vi "MPS_main.vi"() -> ()   [LabVIEW 2021] (continued)
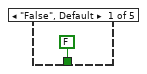
[diagram p2: hidden frame]
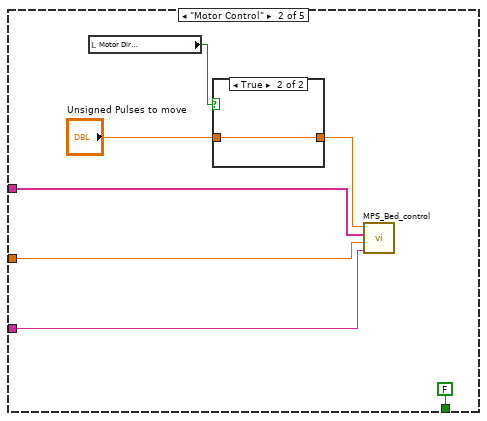
[diagram p3: hidden frame]
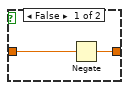
[diagram p4: hidden frame]
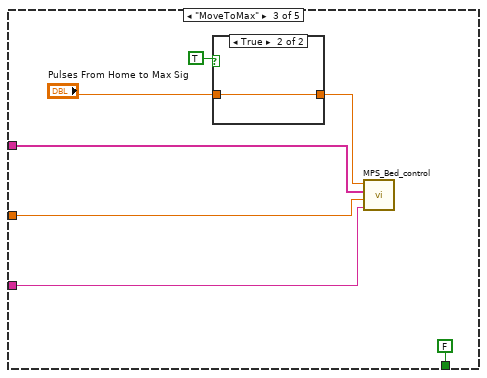
[diagram p5: hidden frame]
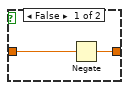
[diagram p6: hidden frame]
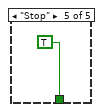
[diagram p7: hidden frame]
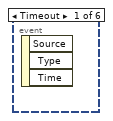
[diagram p8: hidden frame]
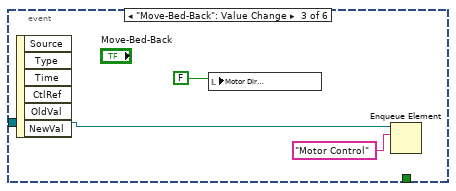
[diagram p9: hidden frame]
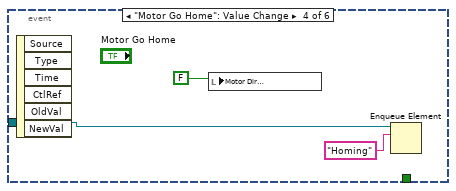
[diagram p10: hidden frame]
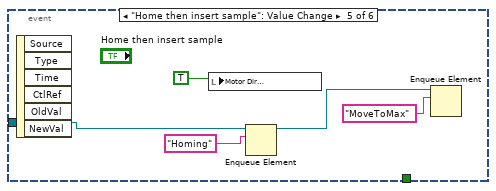
[diagram p11: hidden frame]
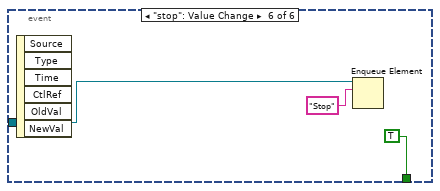
[diagram p12: hidden frame]
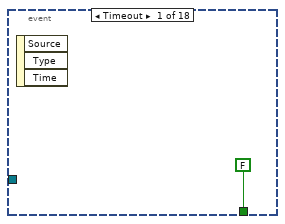
[diagram p13: hidden frame]
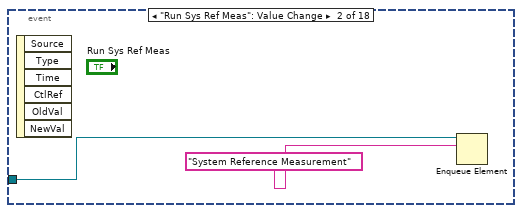
[diagram p14: hidden frame]
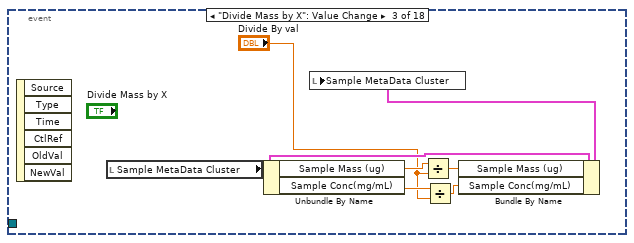
[diagram p15: hidden frame]
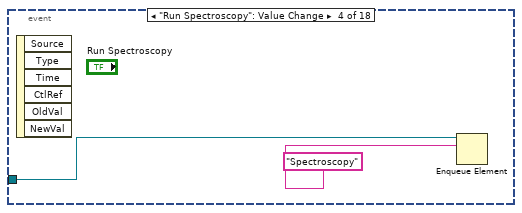
[diagram p16: hidden frame]
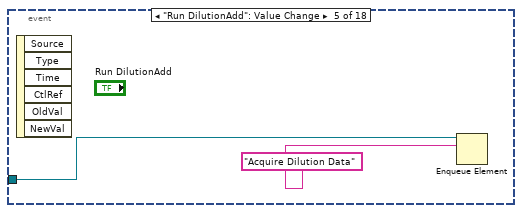
[diagram p17: hidden frame]
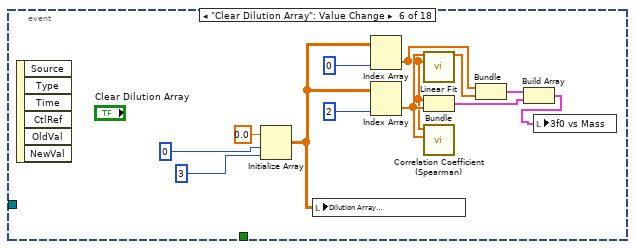
[diagram p18: hidden frame]
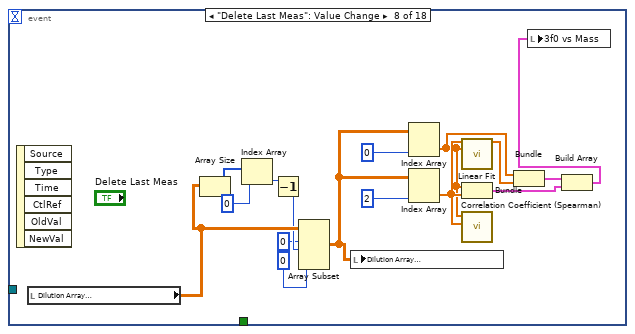
[diagram p19: hidden frame]
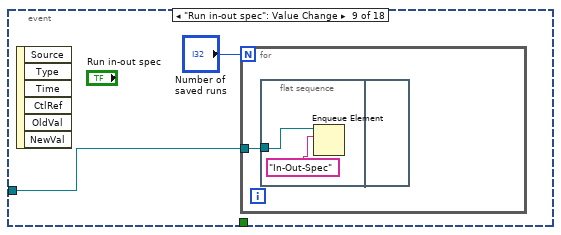
[diagram p20: hidden frame]
            n301 = global read "MPS_global_variables.vi" "Device Name"() -> (w392:tag)
            n302 = call "save_MPS_spectroscopy_hdf.vi"("file path"=w415, "Device Name"=w392, "Phase Rx over time"=w412, "Mag Rx over time"=w413, "TxRx_Params"=w414, "Rx_f0-f8 Units"=w408, "Time Domain Cluster"=w418, "Sample MetaData Cluster"=w399, "Study and Experiment Description"=w400, "Scanner Description"=w401, "Points from home to max"=w402) -> ()  [unwired: 5 in]
          }
        }
        n303 = call <vilib>:"Std Deviation and Variance.vi"("X"=w373) -> ("mean"=→"meanf0":dbl, "standard deviation"=→"standard deviation f0":dbl)  [unwired: 1 in, 1 out]
      }
      frame "Acquire Dilution Data" {
        n304 = Enqueue Element(queue=w532, element="Idle") -> ()  [unwired: 2 in, 3 out]
        n305 = global read "MPS_global_variables.vi" "N Harmonics"() -> (w501:dbl)
        n306 = Initialize Array(0.0 ("element"), 0 ("dimension size"), w501) -> (w529:dbl[][])
        n307 = while {
          shift-right: [w543] -> w525
          shift-left: w529 -> [w544]
          i -> [w542]
          stop <- w535 stop-if-true
          n308 = local read "RxEmptyBore-Spec"() -> (w541:dbl[])
          n309 = call "MPS_Spectroscopy_Core.vi"("EmptyBoreBaseline_Spec"=w541, "ms delay"="ms delay 2", "Spec samples\nto crop"="Spec samples\nto crop 3") -> ("mag f1-f9"=w538:dbl[], "Expected mT Spec Drive"=→"Expected mT Spec Drive 3":dbl, "THD"=→"THD 2":dbl)  [unwired: 2 in, 12 out]
          n310 = Greater Or Equal?(x=w542, y="Num Dil Series Runs") -> (x >= y?=w535:bool)
          n311 = Insert Into Array(array=w544, index (row)=w542, new element=w538) -> (w543:dbl[][])  [unwired: 1 in]
        }
        n312 = local read "Sample MetaData Cluster"() -> (w518:T1)
        n313 = local read "Dilution Array\nConc,f0,f3"() -> (w523:dbl[][])
        n314 = Index Array(array=w525, index (col)=0 ("disabled index (col)")) -> (element=w526:dbl[])  [unwired: 1 in]
        n315 = Index Array(array=w525, index (col)=2 ("index")) -> (element=w528:dbl[])  [unwired: 1 in]
        n316 = Unbundle By Name(w518) -> ("Sample Mass (ug)"=w519:dbl)
        n317 = call <vilib>:"Std Deviation and Variance.vi"("X"=w526) -> ("mean"=w510:dbl)  [unwired: 1 in, 2 out]
        n318 = call <vilib>:"Std Deviation and Variance.vi"("X"=w528) -> ("mean"=w511:dbl)  [unwired: 1 in, 2 out]
        n319 = Array Size(array=w523) -> (size(s)=w522:i32[])
        n320 = Build Array(w519, w510, w511) -> (w517:dbl[])
        n321 = Index Array(array=w522, index=0) -> (element=w521:i32)
        n322 = Insert Into Array(array=w523, index (row)=w521, new element=w517) -> (w515:dbl[][])  [unwired: 1 in]
        n323 = Bundle By Name(cluster=T10 {"slope min"=-inf, "slope max"=inf, "intercept min"=-inf, "intercept max"=inf} ("parameter bounds"), "intercept min"=0.0) -> (w503:T10)
        n324 = local write "Dilution Array\nConc,f0,f3"(w515) -> ()
        n325 = Index Array(array=w515, index (col)=0 ("disabled index (col)")) -> (element=w509:dbl[])  [unwired: 1 in]
        n326 = Index Array(array=w515, index (col)=2 ("disabled index (col)")) -> (element=w507:dbl[])  [unwired: 1 in]
        n327 = call <vilib>:"Linear Fit.vi"("Y"=w507, "X"=w509, "parameter bounds"=w503) -> ("Best Linear Fit"=w513:dbl[])  [unwired: 8 in, 4 out]
        n328 = call <vilib>:"Correlation Coefficient.vi"("Y"=w507, "X"=w509) -> ("r^2"=→"r^2":dbl)  [unwired: 8 in, 1 out]
        n329 = Bundle("Dilution Array\nConc,f0,f3"=w509, "Best Linear Fit"=w513) -> (w505:T17)  [unwired: 1 in]
        n330 = Bundle("Dilution Array\nConc,f0,f3"=w509, "Dilution Array\nConc,f0,f3"=w507) -> (w506:T18)  [unwired: 1 in]
        n331 = Build Array(w505, w506) -> (→"3f0 vs Mass":T6)
      }
      frame "In-Out-Spec" {
        n332 = Enqueue Element(queue=w546, element="Idle") -> ()  [unwired: 2 in, 3 out]
        n333 = flat-sequence {
          tunnel: w545 -> [w785]
          frame #0 {
            w567 = 1 ("index")
            w599 = 0
            n334 = global read "MPS_global_variables.vi" "N Harmonics"() -> (w551:dbl)
            n335 = Multiply(x="Number of cycles", y=2) -> (x*y=w591:i32)
            n336 = Initialize Array(0.0 ("element"), w551, 1 ("dimension size")) -> (w601:dbl[][])
            n337 = Initialize Array(0.0 ("element"), w551, 1 ("dimension size")) -> (w600:dbl[][])
            n338 = Initialize Array(0.0 ("element"), 1 ("dimension size")) -> (w568:dbl[])
            n339 = Initialize Array(0.0 ("element"), 1 ("dimension size")) -> (w587:dbl[])
            n340 = flat-sequence {
              tunnel: w601 -> [w633]
              tunnel: w600 -> [w632]
              tunnel: w599 -> [w631]
              tunnel: w591 -> [w628]
              tunnel: w587 -> [w627]
              tunnel: cluster{"f0":dbl, "df":dbl, "magnitude":dbl[]} {"f0"=0.0, "df"=49.55401387512537, "magnitude"=array[10090 elements]} ("Rx FFT 3") -> [w625]
              tunnel: [w630] -> w620
              tunnel: [w629] -> w619
              tunnel: [w626] -> w618
              tunnel: [w624] -> w617
              tunnel: w568 -> [w623]
              tunnel: [w622] -> w616
              tunnel: [w621] -> w615
              tunnel: [w752] -> w583
              tunnel: [w753] -> w586
              tunnel: [w754] -> w595
              tunnel: [w755] -> w598
              tunnel: w620 -> [w755]
              tunnel: w619 -> [w754]
              tunnel: w618 -> [w753]
              tunnel: w617 -> [w752]
              tunnel: [w750] -> w578
              tunnel: [w749] -> w553
              tunnel: [w748] -> w577
              tunnel: w616 -> [w747]
              tunnel: w615 -> [w746]
              tunnel: [w746] -> w566
              frame #0 {
                n341 = for {
                  N: w628 -> [_]
                  shift-right: [w655] -> w629
                  shift-left: w633 -> [w657]
                  shift-right: [w654] -> w630
                  shift-left: w632 -> [w656]
                  tunnel: w631 -> [_]
                  shift-right: [w645] -> w626
                  shift-left: w627 -> [w646]
                  shift-right: [w639] -> w624
                  shift-left: w625 -> [_]
                  shift-right: [w637] -> w621
                  shift-left: w623 -> [w638]
                  shift-right: [w635] -> w622
                  shift-left: _ -> [_]
                  i -> [w653]
                  n342 = Quotient & Remainder(x=w653, y=2) -> (x-y*floor(x/y)=w643:i32)  [unwired: 1 out]
                  n343 = Decrement(x=w643) -> (x-1=w642:i32)
                  n344 = Equal?(x=w643, y=0) -> (x = y?=w647:bool)
                  n345 = Not(x=w647) -> (.not. x?=w648:bool)
                  n346 = Absolute Value(x=w642) -> (abs(x)=w641:i32)
                  n347 = flat-sequence {
                    tunnel: w657 -> [w670]
                    tunnel: w656 -> [w669]
                    tunnel: [w668] -> w650
                    tunnel: [w667] -> w649
                    tunnel: w648 -> [w666]
                    tunnel: w646 -> [w665]
                    tunnel: w641 -> [w664]
                    tunnel: [w663] -> w644
                    tunnel: [w662] -> w640
                    tunnel: [w661] -> w639
                    tunnel: w638 -> [w660]
                    tunnel: [w659] -> w636
                    tunnel: [w658] -> w634
                    tunnel: [w741] -> w654
                    tunnel: [w742] -> w655
                    tunnel: w650 -> [w742]
                    tunnel: w649 -> [w741]
                    tunnel: w647 -> [w737]
                    tunnel: [w728] -> w645
                    tunnel: w644 -> [w728]
                    tunnel: w640 -> [_]
                    tunnel: [w727] -> w637
                    tunnel: w636 -> [w727]
                    tunnel: [w726] -> w635
                    tunnel: w634 -> [w726]
                    frame #0 {
                      n348 = while {
                        shift-right: [w721] -> w668
                        shift-left: w670 -> [w722]
                        shift-right: [w716] -> w667
                        shift-left: w669 -> [w720]
                        tunnel: w666 -> [w703]
                        tunnel: w664 -> [w699]
                        shift-right: [w698] -> w663
                        shift-left: w665 -> [w700]
                        tunnel: [w694] -> w662
                        tunnel: [w693] -> w661
                        shift-right: [w686] -> w659
                        shift-left: w660 -> [w685]
                        tunnel: [w682] -> w658
                        i -> [w705]
                        stop <- w717 stop-if-true
                        w711 = T15 1 items=["Rectangle"=0, "Hanning"=1, "Hamming"=2, "Blackman-Harris"=3, "Exact Blackman"=4, "Blackman"=5, "Flat Top"=6, "4 Term B-Harris "=7, "7 Term B-Harris"=8, "Low Sidelobe"=9, "Blackman Nuttall"=11, "Triangle"=30, "Bartlett-Hanning"=31, "Bohman"=32, "Parzen"=33, "Welch"=34, "Kaiser"=60, "Dolph-Chebyshev"=61, "Gaussian"=62] ("window")
                        n349 = local write "Bed moving"(FALSE ("Bed moving")) -> ()
                        n350 = global read "MPS_global_variables.vi" "TxRx_Params"() -> (w692:T2)
                        n351 = Greater Or Equal?(x=w705, y="Num acq per\ncycle") -> (x >= y?=w717:bool)
                        n352 = Equal?(x=w705, y=0) -> (x = y?=w702:bool)
                        n353 = Unbundle By Name(w692) -> ("Tx Freq Division Factor"=w691:dbl)
                        n354 = And(x=w702, y=w703) -> (x .and. y?=w688:bool)
                        n355 = local read "RxEmptyBore-Spec"() -> (w715:dbl[])
                        n356 = Multiply(x="Spec drive periods\nto crop_InOut", y=w691) -> (x*y=w682:dbl)
                        n357 = And(x="Reset Baseline\nEach out cycle", y=w688) -> (x .and. y?=w687:bool)
                        n358 = local read "Run number"() -> (w706:i32)
                        n359 = call "MPS_Spectroscopy_Core.vi"("EmptyBoreBaseline_Spec"=w715, "ms delay"="ms delay\nevery Spec", "Spec samples\nto crop"=w682) -> ("Raw Measured"=w701:dbl[], "f0 Complex"=w708:cdb, "phase f1-f9"=w718:dbl[], "TF Corr Rx FFT complex"=w680:T12, "Spec Waveform Baseline Sub"=w673:waveform(dbl), "3f0 Complex"=w710:cdb, "mag f1-f9"=w678:dbl[], "Expected mT Spec Drive"=→"Expected mT Spec Drive 2":dbl, "TF Corrected\nMagnetization over time"=w697:waveform(dbl)[], "Spec Time Domain"=w672:dbl[][], "THD"=→"Drive Imon THD 2":dbl)  [unwired: 2 in, 4 out]
                        n360 = call "TF_Complex_toMagPhase.vi"("TF Corr Rx FFT Mag"=w680) -> ("TF Mag"=→"Rx FFT 2":cluster{"f0":dbl, "df":dbl, "magnitude":dbl[]})  [unwired: 4 in, 6 out]
                        n361 = Increment(x=w706) -> (x+1=w684:i32)
                        n362 = Tick Count (ms)() -> (millisecond timer value=w683:u32)
                        "millisecond timer value" <- w683
                        n363 = case shown="True" w687 {
                          tunnel: w701 -> [_ w723]
                          frame False {
                          }
                          frame True {
                            n364 = local write "RxEmptyBore-Spec"(w723) -> ()
                          }
                        }
                        n365 = local write "Run number"(w684) -> ()
                        n366 = Insert Into Array(array=w722, index (col)=w684, new element=w678) -> (w721:dbl[][])  [unwired: 1 in]
                        n367 = Insert Into Array(array=w720, index (col)=w684, new element=w718) -> (w716:dbl[][])  [unwired: 1 in]
                        n368 = Insert Into Array(array=w685, index=w684, new element=w683) -> (w686:dbl[])
                        n369 = Insert Into Array(array=w700, index=w684, new element=w699) -> (w698:dbl[])
                        n370 = Complex To Polar(r * e^(i*theta)=w708) -> (r=→"f0 over time 2":dbl)  [unwired: 1 out]
                        n371 = Complex To Polar(r * e^(i*theta)=w710) -> (r=w674:dbl, theta=→"3f0 Phase  over time":dbl)
                        n372 = call "NumericArray to WaveformArray.vi"("Array input"=w672, "Ref Waveform"=w673) -> ("Array of waveforms"=→"Spec Time Domain\nInOut":waveform(dbl)[])  [unwired: 9 in]
                        n373 = Index Array(array=w697, index=1) -> (element=w695:waveform(dbl))
                        n374 = Index Array(array=w678, index=1) -> (element=w676:dbl)
                        n375 = Bundle(w676, w674) -> (→"2,3f0 over time":cluster{dbl, dbl})  [unwired: 1 in]
                        n376 = call-poly <vilib>:"FFT Spectrum (Mag-Phase).vi"("window"=w711, "time signal"=w673) -> ("magnitude"=w693:cluster{"f0":dbl, "df":dbl, "magnitude":dbl[]})  [unwired: 5 in, 4 out]
                        n377 = Unbundle By Name(w695) -> ("Y"=w694:dbl[])
                        "Loop Num 2" <- w705
                      }
                    }
                    frame #1 {
                      w734 = 0.0005 ("pulse duration (T/2)")
                      n378 = local write "Bed moving"(TRUE) -> ()
                      n379 = Multiply(x="Pulses in/out", y=w734) -> (x*y=w736:dbl)
                      n380 = case shown="True" w737 {
                        tunnel: [w743 w744] -> w740
                        tunnel: "Pulses in/out" -> [w743 w745]
                        frame False {
                        }
                        frame True {
                          n381 = Negate(x=w745) -> (-x=w744:dbl)
                        }
                      }
                      n382 = local read "Motor speed"() -> (w724:string)
                      n383 = Multiply(x=w736, y=1.0) -> (x*y=w733:dbl)
                      n384 = Multiply(x=w733, y=1.25) -> (x*y=w732:dbl)
                      n385 = call "MPS_Bed_control.vi"("Motor speed"=w724, "pulse duration (T/2)"=w734, "Sequence to run on start up"=string[] ["Move", "Halt"] ("Sequence to run on start up\n 2"), "Signed pulses to move"=w740) -> ()  [unwired: 8 in]
                      n386 = Multiply(x=1000.0, y=w732) -> (x*y=w730:dbl)
                      n387 = Wait (ms)(milliseconds to wait=w730) -> ()  [unwired: 1 out]
                    }
                  }
                }
              }
              frame #1 {
                # "Final Acq.\nwith sample in\nto save time domain"
                n388 = local read "RxEmptyBore-Spec"() -> (w751:dbl[])
                n389 = call "MPS_Spectroscopy_Core.vi"("EmptyBoreBaseline_Spec"=w751, "Spec samples\nto crop"=w747) -> ("Spec Waveform Baseline Sub"=w750:waveform(dbl), "TxIMon cluster"=w749:T13, "TF Corrected\nMagnetization over time"=w748:waveform(dbl)[])  [unwired: 3 in, 12 out]
              }
            }
            n390 = call "get_freq_vector.vi"("FFT magnitude"=w583) -> ("Freq array"=w585:dbl[])  [unwired: 10 in]
            n391 = Unbundle(w553) -> ("output waveform"=w552:waveform(dbl))  [unwired: 1 out]
            n392 = Array Subset(array=w566, index=w567) -> (w563:dbl[])  [unwired: 1 in]
            n393 = Array Subset(array=w586, index=w567) -> (w562:dbl[])  [unwired: 1 in]
            n394 = Array Subset(array=w595, index (row)=0 ("index"), index (col)=1 ("index")) -> (w560:dbl[][])  [unwired: 2 in]
            n395 = Array Subset(array=w598, index (row)=0 ("index"), index (col)=1 ("index")) -> (w561:dbl[][])  [unwired: 2 in]
            n396 = Index Array(array=w577, index=1) -> (element=w575:waveform(dbl))
            n397 = local read "Sample MetaData Cluster"() -> (w557:T1)
            n398 = Bundle By Name(cluster=T11 {"Sample in_vs_Out"=[], "Sample Timing"=[]} ("Sample In Out Cluster"), "Sample in_vs_Out"=w562, "Sample Timing"=w563) -> (w564:T11)
            n399 = call "Process_InOutData.vi"("InOutBool"=w562, "TimeData"=w563, "f0_f9Phase"=w561, "f0_f9Mag"=w560) -> ("SNR"=w556:dbl[][], "Betas"=w559:dbl[][])  [unwired: 2 in, 4 out]
            "Regression\nAmplitudes" <- w559
            "SNR" <- w556
            n400 = global read "MPS_global_variables.vi" "Rx TF File"() -> (w582:string)
            n401 = Unbundle By Name(w578) -> ("Y"=w574:dbl[])
            n402 = Unbundle By Name(w575) -> ("Y"=w572:dbl[])
            n403 = Unbundle By Name(w552) -> ("Y"=w573:dbl[])
            n404 = call "loadTF_resample.vi"("desired freqs"=w585, "mat file name"=w582) -> ("TF units from loaded file"=w579:string, "output TF phase"=w580:dbl[], "output TF mag"=w581:dbl[])  [unwired: 7 in]
            n405 = Unbundle By Name(w557) -> ("Sample Mass (ug)"=w555:dbl)
            n406 = Divide(x=w556, y=w555) -> (x/y=→"SNR per ug":dbl[][])
            n407 = local read "Study and Experiment Description"() -> (w608:T5)
            n408 = local read "Pulses From Home to Max Sig"() -> (w571:dbl)
            n409 = Decrement(x="Plotted harmonic \n(3 = 3f0)") -> (x-1=w548:i32)
            n410 = local read "Sample MetaData Cluster"() -> (w607:T1)
            n411 = local read "Empty Bore-BMon-Spec"() -> (w611:dbl[])
            n412 = Index Array(array=w559, index (row)="Plotted regressor", index (col)=w548) -> (element=→"Regression amplitude over time" →"Most recent amplitude":dbl)
            n413 = local read "Scanner Description"() -> (w609:T4)
            n414 = local read "RxEmptyBore-Spec"() -> (w610:dbl[])
            n415 = Initialize Array(0.0 ("element"), 1 ("dimension size")) -> (w612:dbl[])
            n416 = case shown="True" "Save Spectroscopy 2" {
              tunnel: w610 -> [_ w781]
              tunnel: w611 -> [_ w780]
              tunnel: w607 -> [_ w779]
              tunnel: w608 -> [_ w778]
              tunnel: w609 -> [_ w777]
              tunnel: w612 -> [_ w772]
              tunnel: w560 -> [_ w773]
              tunnel: w561 -> [_ w774]
              tunnel: w581 -> [_ w771]
              tunnel: w580 -> [_ w769]
              tunnel: w579 -> [_ w768]
              tunnel: w574 -> [_ w767]
              tunnel: w573 -> [_ w757]
              tunnel: w572 -> [_ w766]
              tunnel: w571 -> [_ w764]
              tunnel: w564 -> [_ w758]
              frame False {
              }
              frame True {
                w760 = u16 2 items=["Spec.", "Mag.", "In Out Spec"] ("Ring")
                n417 = Bundle By Name(cluster=T9 {"Drive IMon"=array[500000 elements], "Rx Time Domain"=array[500000 elements], "Rx Empty Bore"=array[500000 elements], "BMon"=array[500000 elements], "Bias IMon"=array[500000 elements], "TF-Corr-MagOverTime"=[], "Interpolated Rx TF-Mag"=[], "Interpolated Rx TF-Phase"=[]} ("Time Domain Cluster 2"), "Drive IMon"=w757, "Rx Time Domain"=w767, "Rx Empty Bore"=w781, "BMon"=w780, "Bias IMon"=w772, "TF-Corr-MagOverTime"=w766, "Interpolated Rx TF-Mag"=w771, "Interpolated Rx TF-Phase"=w769) -> (w765:T9)
                n418 = local read "Sample MetaData Cluster"() -> (w762:T1)
                n419 = local read "name identifier"() -> (w763:string)
                n420 = local read "Base path"() -> (w761:path)
                n421 = global read "MPS_global_variables.vi" "TxRx_Params"() -> (w775:T2)
                n422 = call "Spectrometer_File_Naming.vi"("Description"=w763, "Sample MetaData Cluster"=w762, "Ring"=w760) -> ("Output Name"=w759:string)  [unwired: 8 in]
                n423 = local write "Recent File Name"(w759) -> ()
                n424 = call "file_path.vi"("name identifier"=w759, "Base path"=w761) -> ("HDF path"=w776:path)  [unwired: 7 in, 2 out]
                n425 = global read "MPS_global_variables.vi" "Device Name"() -> (w756:tag)
                n426 = call "save_MPS_spectroscopy_hdf.vi"("file path"=w776, "Device Name"=w756, "Phase Rx over time"=w774, "Mag Rx over time"=w773, "TxRx_Params"=w775, "Rx_f0-f8 Units"=w768, "Time Domain Cluster"=w765, "Sample MetaData Cluster"=w779, "Study and Experiment Description"=w778, "Sample In Out Cluster"=w758, "Scanner Description"=w777, "Points from home to max"=w764) -> ()  [unwired: 4 in]
              }
            }
            "Run number" <- w599
          }
          frame #1 {
            n427 = Wait (ms)(milliseconds to wait=u32 5) -> ()  [unwired: 1 out]
          }
          frame #2 {
            n428 = Wait (ms)(milliseconds to wait=u32 13000) -> ()  [unwired: 1 out]
            n429 = Enqueue Element(queue=w785, element="Homing") -> (queue out=w787:refnum<queue>)  [unwired: 2 in, 2 out]
            n430 = Enqueue Element(queue=w787, element="MoveToMax") -> ()  [unwired: 2 in, 3 out]
          }
        }
      }
      frame "Update Meta" {
      }
      frame "Magnetometry" {
        w811 = T15 1 items=["Rectangle"=0, "Hanning"=1, "Hamming"=2, "Blackman-Harris"=3, "Exact Blackman"=4, "Blackman"=5, "Flat Top"=6, "4 Term B-Harris "=7, "7 Term B-Harris"=8, "Low Sidelobe"=9, "Blackman Nuttall"=11, "Triangle"=30, "Bartlett-Hanning"=31, "Bohman"=32, "Parzen"=33, "Welch"=34, "Kaiser"=60, "Dolph-Chebyshev"=61, "Gaussian"=62] ("window")
        n431 = local read "EmptyBoreBaseline_Mag"() -> (w802:dbl[])
        n432 = Array Size(array=w802) -> (size(s)=w798:i32)
        n433 = Multiply(x="Num Mag Avgs", y=2) -> (x*y=w792:i32)
        n434 = Initialize Array(0.0 ("element"), w798, "Num Mag Avgs") -> (w803:dbl[][])
        n435 = for {
          N: w792 -> [_]
          tunnel: [w842] -> w790
          tunnel: [w841] -> w812
          tunnel: [w840] -> w795
          shift-right: [w838] -> w800
          shift-left: w803 -> [w839]
          i -> [w832]
          n436 = Quotient & Remainder(x=w832, y=2) -> (x-y*floor(x/y)=w835:i32, floor(x/y)=w831:i32)
          n437 = Equal?(x=w835, y=0) -> (x = y?=w827:bool)
          n438 = Not(x=w827) -> (.not. x?=w828:bool)
          "Sample Out" <- w828
          n439 = flat-sequence {
            tunnel: [w858] -> w842
            tunnel: [w846] -> w840
            tunnel: w839 -> [w852]
            tunnel: [w856] -> w837
            tunnel: [w850] -> w836
            tunnel: w828 -> [w853]
            tunnel: w831 -> [w849]
            tunnel: w827 -> [w844]
            tunnel: w837 -> [w885]
            tunnel: w836 -> [w884]
            tunnel: w827 -> [w876]
            tunnel: [w885] -> w830
            tunnel: [w884] -> w829
            tunnel: [w890] -> w838
            tunnel: [w891] -> w841
            tunnel: w830 -> [w891]
            tunnel: w829 -> [w890]
            frame #0 {
              n440 = local read "EmptyBoreBaseline_Mag_BMon"() -> (w859:dbl[])
              n441 = local write "Bed moving"(FALSE) -> ()
              n442 = local read "EmptyBoreBaseline_Mag"() -> (w860:dbl[])
              n443 = call "MPS_Mag_Core.vi"("EmptyBoreBaseline_Mag_BMon"=w859, "EmptyBoreBaseline_Mag"=w860) -> ("Samples Per Acquisition"=w855:dbl, "Drive IMon"=w857:waveform(dbl), "Susceptibility Curves"=w843:cluster{"Y":dbl[], "Y":dbl[]}[], "Rx Smooth"=→"Rx Smooth":dbl[], "Bias Current"=w858:waveform(dbl), "Rx_Raw"=w847:waveform(dbl), "RxBaselineSub"=w846:waveform(dbl))  [unwired: 5 in, 2 out]
              n444 = case shown="True" w844 {
                tunnel: w846 -> [_ w862]
                tunnel: w843 -> [_ w861]
                frame False {
                }
                frame True {
                  n445 = call "MPS_Mag_Proc_Spectrogram.vi"("Signal"=w862) -> ("Sensitivity profile"=→"Sensitivity profile":dbl[][])  [unwired: 9 in, 1 out]
                  "Susceptibility Curves" <- w861
                }
              }
              n446 = Unbundle By Name(w846) -> ("Y"=w845:dbl[])
              n447 = Unbundle By Name(w847) -> ("Y"=w851:dbl[])
              n448 = local write "Samples Per Acquisition"(w855) -> ()
              n449 = case shown="False" w853 {
                tunnel: w852 -> [w867 w869]
                tunnel: w851 -> [_ w868]
                tunnel: [w866 w869] -> w850
                tunnel: w849 -> [w865 _]
                tunnel: w845 -> [w864 _]
                frame False {
                  n450 = Replace Array Subset(array=w867, new element=w864, index (col)=w865) -> (w866:dbl[][])  [unwired: 1 in]
                  "RunNum" <- w865
                }
                frame True {
                  n451 = local write "EmptyBoreBaseline_Mag"(w868) -> ()
                }
              }
              n452 = Unbundle By Name(w857) -> ("Y"=w856:dbl[])
            }
            frame #1 {
              w874 = 0.0005 ("pulse duration (T/2)")
              n453 = local write "Bed moving"(TRUE) -> ()
              n454 = local read "Motor speed"() -> (w870:string)
              n455 = case shown="True" w876 {
                tunnel: [w886 w887] -> w878
                tunnel: "Pulses in/out 2" -> [w886 w888]
                frame False {
                }
                frame True {
                  n456 = Negate(x=w888) -> (-x=w887:dbl)
                }
              }
              n457 = Multiply(x="Pulses in/out 2", y=w874) -> (x*y=w879:dbl)
              n458 = Multiply(x=w879, y=1.0) -> (x*y=w880:dbl)
              n459 = Multiply(x=w880, y=1.25) -> (x*y=w881:dbl)
              n460 = call "MPS_Bed_control.vi"("Motor speed"=w870, "pulse duration (T/2)"=w874, "Sequence to run on start up"=string[] ["Move", "Halt"] ("Sequence to run on start up\n 2"), "Signed pulses to move"=w878) -> ()  [unwired: 8 in]
              n461 = Multiply(x=1000.0, y=w881) -> (x*y=w882:dbl)
              n462 = Wait (ms)(milliseconds to wait=w882) -> ()  [unwired: 1 out]
            }
            frame #2 {
              n463 = Wait (ms)(milliseconds to wait="ms delay each run") -> ()  [unwired: 1 out]
            }
          }
        }
        n464 = Initialize Array(0.0 ("element"), w798) -> (w797:dbl[])
        n465 = for {
          N: "Num Mag Avgs" -> [_]
          shift-right: [w823] -> w796
          shift-left: w797 -> [w824]
          shift-right: [w822] -> _
          shift-left: w800 -> [w822]
          i -> [w826]
          n466 = Index Array(array=w822, index (col)=w826) -> (element=w825:dbl[])  [unwired: 1 in]
          n467 = Add(x=w825, y=w824) -> (x+y=w823:dbl[])
        }
        n468 = call-poly <vilib>:"FFT Spectrum (Mag-Phase).vi"("window"=w811, "time signal"=w795) -> ("magnitude"=w809:cluster{"f0":dbl, "df":dbl, "magnitude":dbl[]})  [unwired: 5 in, 4 out]
        n469 = call "get_freq_vector.vi"("FFT magnitude"=w809) -> ("Freq array"=w810:dbl[])  [unwired: 10 in]
        n470 = global read "MPS_global_variables.vi" "Rx TF File"() -> (w808:string)
        n471 = Divide(x=w796, y="Num Mag Avgs") -> (x/y=w791:dbl[])
        n472 = Unbundle By Name(w790) -> ("Y"=w813:dbl[])
        n473 = call "loadTF_resample.vi"("desired freqs"=w810, "mat file name"=w808) -> ("TF units from loaded file"=w805:string, "output TF phase"=w807:dbl[], "output TF mag"=w806:dbl[])  [unwired: 7 in]
        n474 = local read "Study and Experiment Description"() -> (w816:T5)
        n475 = local read "EmptyBoreBaseline_Mag_BMon"() -> (w818:dbl[])
        n476 = local read "Pulses From Home to Max Sig"() -> (w804:dbl)
        n477 = local read "Sample MetaData Cluster"() -> (w817:T1)
        n478 = local read "EmptyBoreBaseline_Mag"() -> (w819:dbl[])
        n479 = Bundle By Name(cluster=w790, "Y"=w791) -> (w789:waveform(dbl))
        n480 = local read "Scanner Description"() -> (w815:T4)
        n481 = call "MPS_Mag_Proc_Spectrogram.vi"("Signal"=w789) -> ("Sensitivity profile"=→"Sensitivity profile 2":dbl[][])  [unwired: 9 in, 1 out]
        n482 = case shown="True" "Save Mag data" {
          tunnel: w818 -> [_ w916]
          tunnel: w817 -> [_ w915]
          tunnel: w816 -> [_ w914]
          tunnel: w815 -> [_ w913]
          tunnel: w819 -> [_ w911]
          tunnel: w813 -> [_ w907]
          tunnel: w812 -> [_ w906]
          tunnel: w807 -> [_ w904]
          tunnel: w806 -> [_ w903]
          tunnel: w805 -> [_ w902]
          tunnel: w804 -> [_ w899]
          tunnel: w791 -> [_ w893]
          frame False {
          }
          frame True {
            w896 = u16 1 items=["Spec.", "Mag.", "In Out Spec"] ("Ring")
            n483 = Bundle By Name(cluster=T9 {"Drive IMon"=array[500000 elements], "Rx Time Domain"=array[500000 elements], "Rx Empty Bore"=array[500000 elements], "BMon"=array[500000 elements], "Bias IMon"=array[500000 elements], "TF-Corr-MagOverTime"=[], "Interpolated Rx TF-Mag"=[], "Interpolated Rx TF-Phase"=[]} ("Time Domain Cluster 3"), "Drive IMon"=w906, "Rx Time Domain"=w893, "Rx Empty Bore"=w911, "BMon"=w916, "Bias IMon"=w907, "TF-Corr-MagOverTime"=dbl[] [], "Interpolated Rx TF-Mag"=w903, "Interpolated Rx TF-Phase"=w904) -> (w901:T9)
            n484 = local read "Sample MetaData Cluster"() -> (w898:T1)
            n485 = local read "name identifier"() -> (w897:string)
            n486 = local read "Base path"() -> (w895:path)
            n487 = global read "MPS_global_variables.vi" "TxRx_Params"() -> (w909:T2)
            n488 = call "Spectrometer_File_Naming.vi"("Description"=w897, "Sample MetaData Cluster"=w898, "Ring"=w896) -> ("Output Name"=w894:string)  [unwired: 8 in]
            n489 = local write "Recent File Name"(w894) -> ()
            n490 = call "file_path.vi"("name identifier"=w894, "Base path"=w895) -> ("HDF path"=w912:path)  [unwired: 7 in, 2 out]
            n491 = global read "MPS_global_variables.vi" "Device Name"() -> (w892:tag)
            n492 = Initialize Array(0.0 ("element")) -> (w908:dbl[][])  [unwired: 2 in]
            n493 = call "save_MPS_spectroscopy_hdf.vi"("file path"=w912, "Device Name"=w892, "Phase Rx over time"=w908, "Mag Rx over time"=w908, "TxRx_Params"=w909, "Rx_f0-f8 Units"=w902, "Time Domain Cluster"=w901, "Sample MetaData Cluster"=w915, "Study and Experiment Description"=w914, "Scanner Description"=w913, "Points from home to max"=w899) -> ()  [unwired: 5 in]
          }
        }
        n494 = Enqueue Element(queue=w820, element="Idle") -> ()  [unwired: 2 in, 3 out]
      }
      frame "Acquire Empty Bore" {
        n495 = Enqueue Element(queue=w917, element="Idle") -> ()  [unwired: 2 in, 3 out]
        n496 = stacked-sequence {
          frame #0 {
            # "Data queue"
            # "Data queue"
            n497 = global read "MPS_global_variables.vi" "TxRx_Params"() -> (w928:T2)
            n498 = Unbundle By Name(w928) -> ("Tx cycles\nSpectroscopy"=w924:dbl, "sample rate"=w927:dbl, "Tx freq"=w926:dbl)
            n499 = Obtain Queue(element data type=waveform(dbl) {"t0"=timestamp(0 s since 1904-01-01), "dt"=1.0, "Y"=[]} ("Waveform")) -> (queue out=w929:refnum<queue>)  [unwired: 4 in, 2 out]
            n500 = Obtain Queue(element data type=waveform(dbl) {"t0"=timestamp(0 s since 1904-01-01), "dt"=1.0, "Y"=[]} ("Waveform")) -> (queue out=w921:refnum<queue>)  [unwired: 4 in, 2 out]
            n501 = Divide(x=w927, y=w926) -> (x/y=w925:dbl)
            n502 = Multiply(x=w924, y=w925) -> (x*y=w923:dbl)
            n503 = flat-sequence {
              tunnel: w929 -> [w931]
              tunnel: w923 -> [w934]
              tunnel: [w933] -> w922
              tunnel: w922 -> [w945]
              tunnel: w921 -> [w942]
              frame #0 {
                w936 = T15 1 items=["Rectangle"=0, "Hanning"=1, "Hamming"=2, "Blackman-Harris"=3, "Exact Blackman"=4, "Blackman"=5, "Flat Top"=6, "4 Term B-Harris "=7, "7 Term B-Harris"=8, "Low Sidelobe"=9, "Blackman Nuttall"=11, "Triangle"=30, "Bartlett-Hanning"=31, "Bohman"=32, "Parzen"=33, "Welch"=34, "Kaiser"=60, "Dolph-Chebyshev"=61, "Gaussian"=62] ("window")
                n504 = call <extravilib>:"Write.vi"("element"=1 ("number of readouts")) -> ("channel"=w939:T16)  [unwired: 1 out]
                n505 = Dequeue Element(queue=w931) -> (element=w930:waveform(dbl))  [unwired: 2 in, 3 out]
                n506 = call-poly <vilib>:"FFT Spectrum (Mag-Phase).vi"("window"=w936, "time signal"=w930) -> ("magnitude"=w935:cluster{"f0":dbl, "df":dbl, "magnitude":dbl[]})  [unwired: 5 in, 4 out]
                n507 = Round To Nearest(number=w934) -> (nearest integer value=w933:dbl)
                n508 = Unbundle By Name(w930) -> ("Y"=w937:dbl[])
                "EmptyBoreBaseline_Spec" <- w937
                "RxEmptyBore-Spec" <- w937
                n509 = call "MPS_transmit_receive.vi"("samples per readout"=w933, "Use Bias?"=FALSE, "InputChans"=enum16{"Rx", "BiasIMon", "TxIMon", "BMon"}."Rx", "channel input for max readouts"=w939, "Measurement Queue"=w931) -> ()  [unwired: 7 in]
                n510 = local write "Samples Per Acquisition"(w933) -> ()
                n511 = local write "EmptyBoreBaseline_Spec"(w937) -> ()
                n512 = Complex To Polar(r * e^(i*theta)=w935) -> ()  [unwired: 2 out]
              }
              frame #1 {
                n513 = Round To Nearest(number=w945) -> (nearest integer value=w948:dbl)
                n514 = call <extravilib>:"Write.vi"("element"=1 ("number of readouts")) -> ("channel"=w949:T16)  [unwired: 1 out]
                n515 = Dequeue Element(queue=w942) -> (element=w944:waveform(dbl))  [unwired: 2 in, 3 out]
                n516 = call "MPS_transmit_receive.vi"("samples per readout"=w948, "Use Bias?"=TRUE, "InputChans"=enum16{"Rx", "BiasIMon", "TxIMon", "BMon"}."BMon", "channel input for max readouts"=w949, "Measurement Queue"=w942) -> ()  [unwired: 7 in]
                n517 = Unbundle By Name(w944) -> ("Y"=→"Empty Bore-BMon-Spec" →"Bmon plot":dbl[])  [unwired: 1 out]
              }
            }
          }
          frame #1 {
            n518 = Wait (ms)(milliseconds to wait=u32 100) -> ()  [unwired: 1 out]
          }
          frame #2 {
            # "Data queue"
            # "Data queue"
            n519 = global read "MPS_global_variables.vi" "TxRx_Params"() -> (w960:T2)
            n520 = Unbundle By Name(w960) -> ("Bias Periods\nMagnetometry"=w956:dbl, "sample rate"=w959:dbl, "Bias freq"=w958:dbl)
            n521 = Obtain Queue(element data type=waveform(dbl) {"t0"=timestamp(0 s since 1904-01-01), "dt"=1.0, "Y"=[]} ("Waveform")) -> (queue out=w961:refnum<queue>)  [unwired: 4 in, 2 out]
            n522 = Obtain Queue(element data type=waveform(dbl) {"t0"=timestamp(0 s since 1904-01-01), "dt"=1.0, "Y"=[]} ("Waveform")) -> (queue out=w954:refnum<queue>)  [unwired: 4 in, 2 out]
            n523 = Divide(x=w959, y=w958) -> (x/y=w957:dbl)
            n524 = Multiply(x=w956, y=w957) -> (x*y=w955:dbl)
            n525 = flat-sequence {
              tunnel: w961 -> [w963]
              tunnel: w955 -> [w966]
              tunnel: [w966] -> w953
              tunnel: w954 -> [w972]
              tunnel: w953 -> [w974]
              frame #0 {
                n526 = Dequeue Element(queue=w963) -> (element=w964:waveform(dbl))  [unwired: 2 in, 3 out]
                "RxEmptyBore-Mag" <- w964
                n527 = Round To Nearest(number=w966) -> (nearest integer value=w968:dbl)
                n528 = call <extravilib>:"Write.vi"("element"=1 ("number of readouts")) -> ("channel"=w969:T16)  [unwired: 1 out]
                n529 = Unbundle By Name(w964) -> ("Y"=w965:dbl[])
                "EmptyBoreBaseline_Mag" <- w965
                n530 = call "MPS_transmit_receive.vi"("samples per readout"=w968, "Use Bias?"=TRUE, "InputChans"=enum16{"Rx", "BiasIMon", "TxIMon", "BMon"}."Rx", "channel input for max readouts"=w969, "Measurement Queue"=w963) -> ()  [unwired: 7 in]
                n531 = local write "Samples Per Acquisition"(w968) -> ()
                n532 = local write "EmptyBoreBaseline_Mag"(w965) -> ()
              }
              frame #1 {
                (unwired) FALSE ("T=DriveMon \nF=BMon")
                n533 = call <extravilib>:"Write.vi"("element"=1 ("number of readouts")) -> ("channel"=w976:T16)  [unwired: 1 out]
                n534 = Dequeue Element(queue=w972) -> (element=w973:waveform(dbl))  [unwired: 2 in, 3 out]
                n535 = Round To Nearest(number=w974) -> (nearest integer value=w977:dbl)
                n536 = Unbundle By Name(w973) -> ("Y"=w978:dbl[])
                "EmptyBoreBaseline_Mag_BMon" <- w978
                n537 = call "MPS_transmit_receive.vi"("samples per readout"=w977, "Use Bias?"=TRUE, "InputChans"=enum16{"Rx", "BiasIMon", "TxIMon", "BMon"}."BMon", "channel input for max readouts"=w976, "Measurement Queue"=w972) -> ()  [unwired: 7 in]
                n538 = local write "Samples Per Acquisition"(w977) -> ()
                n539 = local write "EmptyBoreBaseline_Mag_BMon"(w978) -> ()
              }
            }
          }
        }
      }
      frame "Zero Baseline" {
        n540 = Enqueue Element(queue=w981, element="Idle") -> ()  [unwired: 2 in, 3 out]
        n541 = local read "RxEmptyBore-Spec"() -> (w987:dbl[])
        n542 = local read "RxEmptyBore-Mag"() -> (w984:waveform(dbl))
        n543 = Multiply(x=w987, y=0.0) -> (x*y=w986:dbl[])
        n544 = Multiply(x=w984, y=0.0) -> (x*y=w985:waveform(dbl))
        n545 = local write "RxEmptyBore-Spec"(w986) -> ()
        n546 = local write "RxEmptyBore-Mag"(w985) -> ()
      }
      frame "Halt" {
      }
    }
  }
  n547 = while {
    tunnel: w1 -> [w990]
    stop <- w989 stop-if-true
    n548 = event shown="[1] \"Move-Bed-Fwd\": Value Change" {
      selector: _ -> [_ _ _ _ _ _]
      dyn-events: _ -> [_ _ _ _ _ _]
      timeout: _ -> [_ _ _ _ _ _]
      tunnel: w990 -> [_ w991 w994 w997 w1002 w1005]
      tunnel: [_ _ _ _ _ TRUE] -> w989
      event Timeout {
        n549 = event-data() -> ()  [unwired: 1 in, 3 out]
      }
      event "Move-Bed-Fwd": Value Change {
        n550 = event-data() -> ()  [unwired: 1 in, 6 out]
        n551 = local write "Motor Dir\nT=Fwd"(TRUE) -> ()
        n552 = Enqueue Element(queue=w991, element="Motor Control") -> ()  [unwired: 2 in, 3 out]
      }
      event "Move-Bed-Back": Value Change {
        n553 = event-data() -> ()  [unwired: 1 in, 6 out]
        n554 = local write "Motor Dir\nT=Fwd"(FALSE) -> ()
        n555 = Enqueue Element(queue=w994, element="Motor Control") -> ()  [unwired: 2 in, 3 out]
      }
      event "Motor Go Home": Value Change {
        n556 = event-data() -> ()  [unwired: 1 in, 6 out]
        n557 = local write "Motor Dir\nT=Fwd"(FALSE) -> ()
        n558 = Enqueue Element(queue=w997, element="Homing") -> ()  [unwired: 2 in, 3 out]
      }
      event "Home then insert sample": Value Change {
        n559 = event-data() -> ()  [unwired: 1 in, 6 out]
        n560 = local write "Motor Dir\nT=Fwd"(TRUE) -> ()
        n561 = Enqueue Element(queue=w1002, element="Homing") -> (queue out=w1000:refnum<queue>)  [unwired: 2 in, 2 out]
        n562 = Enqueue Element(queue=w1000, element="MoveToMax") -> ()  [unwired: 2 in, 3 out]
      }
      event "stop": Value Change {
        n563 = event-data() -> ()  [unwired: 1 in, 6 out]
        n564 = Enqueue Element(queue=w1005, element="Stop") -> ()  [unwired: 2 in, 3 out]
      }
    }
  }
  n565 = while {
    tunnel: w1 -> [w1012]
    stop <- w1011 stop-if-true
    n566 = Dequeue Element(queue=w1012) -> (element=w1013:string)  [unwired: 2 in, 3 out]
    "Current Motor State" <- w1013
    n567 = case shown="\"Homing\"" w1013 {
      tunnel: [FALSE FALSE FALSE FALSE TRUE] -> w1011
      tunnel: "Sequence to run on start up" -> [_ w1017 w1028 _ _]
      tunnel: "Motor speed" -> [_ w1016 w1026 _ _]
      tunnel: "pulse duration (T/2)" -> [_ w1015 w1027 _ _]
      frame "False", Default {
      }
      frame "Motor Control" {
        n568 = local read "Motor Dir\nT=Fwd"() -> (w1019:bool)
        n569 = case shown="True" w1019 {
          tunnel: [w1022 w1024] -> w1020
          tunnel: "Unsigned Pulses to move" -> [w1023 w1024]
          frame False {
            n570 = Negate(x=w1023) -> (-x=w1022:dbl)
          }
          frame True {
          }
        }
        n571 = call "MPS_Bed_control.vi"("Motor speed"=w1016, "pulse duration (T/2)"=w1015, "Sequence to run on start up"=w1017, "Signed pulses to move"=w1020) -> ()  [unwired: 8 in]
      }
      frame "MoveToMax" {
        n572 = case shown="True" TRUE {
          tunnel: [w1032 w1034] -> w1031
          tunnel: "Pulses From Home to Max Sig" -> [w1033 w1034]
          frame False {
            n573 = Negate(x=w1033) -> (-x=w1032:dbl)
          }
          frame True {
          }
        }
        n574 = call "MPS_Bed_control.vi"("Motor speed"=w1026, "pulse duration (T/2)"=w1027, "Sequence to run on start up"=w1028, "Signed pulses to move"=w1031) -> ()  [unwired: 8 in]
      }
      frame "Homing" {
        n575 = flat-sequence {
          frame #0 {
            n576 = local read "pulse duration (T/2)"() -> (w1037:dbl)
            n577 = local read "Motor speed"() -> (w1036:string)
            n578 = call "MPS_Bed_control.vi"("Motor speed"=w1036, "pulse duration (T/2)"=w1037, "Sequence to run on start up"=string[] ["Homing parameters", "Move", "Post homing", "Halt"]) -> ()  [unwired: 9 in]
          }
          frame #1 {
            n579 = local read "Sequence to run on start up"() -> (w1042:string[])
            n580 = local read "pulse duration (T/2)"() -> (w1041:dbl)
            n581 = local read "Motor speed"() -> (w1040:string)
            n582 = call "MPS_Bed_control.vi"("Motor speed"=w1040, "pulse duration (T/2)"=w1041, "Sequence to run on start up"=w1042, "Signed pulses to move"="Pulses to move fwd after homing") -> ()  [unwired: 8 in]
          }
        }
      }
      frame "Stop" {
      }
    }
  }
  n583 = local write "Main loop has stopped"(w12) -> ()
  "Main loop has stopped" <- FALSE ("Main loop has stopped")
